vi "IMAQdx_AbsImage_Flea3_v4.7.vi"() -> ()   [LabVIEW 2013] (continued)
0\tVimaging\t0\t0\t1\t0\t1\t1\t0\tbMOTpow(0.5)\tProbePow\t0\tXshimrMOT\tYshimrMOT\tZshimVar\tODTpowZ(DipPowZ)\tVimaging\t0\t0\tHimaging\t0\t0\t0\t0\t0\t0\t0\t0\t0\t0\t0\t0\t0\t0\trMOTdelta(-(rMOTstirDetI +stirWidthF/2))\tODTpowBlue(0)\tODTpowXY(DipPowCr)\tvarWaveP2\tProbePow2\tAmp688(depumpPow)\trMOTpow3\tODTpowX(DipPowX2)\tfreq\tHeatingAmp\t0\tSine\tDetuning\tsingleFreqDet +20\tDoppCoolDet-DoppCoolSweep\tdopCoolT*1000\tDetuning\tsingleFreqStirDet + 20\tsingleFreqStirDet + SFramp + SFramp2\tloadT*1000\tBlueBN\tBlueLaserProbeBN\tSSteckBN\tShortSteckDDS\tPixisPos(TOF)\tCycle Wait for Move\t0\t0\t0\t0\t0\t0\t0\t0\t0\t0\t0\t0\t0\t0\t0\t0\t0\t0\t0\t0\t0\t0\t0\t0\r\narm DIP FLEA\t\tRamp\t1\tcameraArmT\t0\t0\t0\t0\t0\t0\t0\t0\t0\t0\t0\t0\t0\t0\t0\t0\t0\t0\t0\t0\t0\t0\t0\t0\t0\t1\t1\t0\t0\t0\t1\t0\t0\tplus_zman\tminus_zman\tcompensation\trMOTcurrF\trMOTpow3\tcombAmplitude(combWidthF)\trMOTdelta(-(rMOTbroadDetuningF +combWidthF/2))\tODTpowHLat(DipPowHLat)\t0\tVimaging\t0\t0\t0\t0\t1\t0\t0\tbMOTpow(0.5)\tProbePow\t0\tXshimrMOT\tYshimrMOT\tZshimVar\tODTpowZ(DipPowZ3)\tVimaging\t0\t0\tHimaging\t0\t0\t0\t0\t0\t0\t0\t0\t0\t0\t0\t0\t0\t0\trMOTdelta(-(rMOTstirDetI +stirWidthF/2))\tODTpowBlue(0)\tODTpowXY(DipPowCrTOF)\tvarWaveP1\tProbePow2\tAmp688(depumpPow)\trMOTpow3\tODTpowX(DipPowXTOF)\tfreq\tHeatingAmp\t0\tSine\tDetuning\tsingleFreqDet +20\tDoppCoolDet-DoppCoolSweep\tdopCoolT*1000\tDetuning\tsingleFreqStirDet + 20\tsingleFreqStirDet + SFramp + SFramp2\tloadT*1000\tBlueBN\tBlueLaserProbeBN\tSSteckBN\tShortSteckDDS\tPixisPos(TOF)\tCycle Wait for Move\t0\t0\t0\t0\t0\t0\t0\t0\t0\t0\t0\t0\t0\t0\t0\t0\t0\t0\t0\t0\t0\t0\t0\t0\r\narm BEC FLEA\t\tRamp\t0\tcameraArmT\t1\t1\t1\t1\t1\t1\t0\t0\t0\t0\t0\t0\t0\t0\t0\t0\t0\t0\t0\t0\t0\t0\t0\t0\t0\t1\t1\t0\t0\t0\t1\t0\t0\tplus_zman\tminus_zman\tcompensation\trMOTcurrF\trMOTpow3\tcombAmplitude(combWidthF)\trMOTdelta(-(rMOTbroadDetuningF +combWidthF/2))\tODTpowHLat(DipPowHLat)\t0\tVimaging\t0\t0\t0\t0\t1\t0\t0\tbMOTpow(0.5)\tProbePow\t0\tXshimrMOT\tYshimrMOT\tZshimVar\tODTpowZ(DipPowZ3)\tVimaging\t0\t0\tHimaging\t0\t0\t0\t0\t0\t0\t0\t0\t0\t0\t0\t0\t0\t0\trMOTdelta(-(rMOTstirDetI +stirWidthF/2))\tODTpowBlue(BlueDipPow)\tExpFinal(tEvap1,ODTpowXY(DipPowCr2),ODTpowXY(DipPowCr3),tau)\tvarWaveP1\tProbePow2\tAmp688(depumpPow)\trMOTpow3\tExpFinal(tEvap1,ODTpowX(DipPowX2),ODTpowX(DipPowX3),tau)\tfreq\tHeatingAmp\t0\tSine\tDetuning\tsingleFreqDet +20\tDoppCoolDet-DoppCoolSweep\tdopCoolT*1000\tDetuning\tsingleFreqStirDet + 20\tsingleFreqStirDet + SFramp + SFramp2\tloadT*1000\tBlueBN\tBlueLaserProbeBN\tSSteckBN\tShortSteckDDS\tPixisPos(TOF)\tCycle Wait for Move\t0\t0\t0\t0\t0\t0\t0\t0\t0\t0\t0\t0\t0\t0\t0\t0\t0\t0\t0\t0\t0\t0\t0\t0\r\natom img\t\tRamp\t1\texposureT\t0\t0\t0\t0\t0\t0\t0\t0\t1\t0\t0\t0\t0\t1\t0\t0\t0\t0\t1\t0\t0\t0\t0\t0\t0\t1\t1\t0\t0\t0\t1\t0\t0\tplus_zman\tminus_zman\tcompensation\trMOTcurrF\trMOTpow3\tcombAmplitude(combWidthF)\trMOTdelta(-(rMOTbroadDetuningF +combWidthF/2))\tODTpowHLat(DipPowHLat)\t0\tVimaging\t0\t0\t0\t0\t0\t0\t0\tbMOTpow(0.5)\tProbePow\t0\tXshimrMOT\tYshimrMOT\tZshimVar\tODTpowZ(DipPowZ)\tVimaging\t0\t0\tHimaging\t0\t0\t0\t0\t0\t0\t0\t0\t0\t0\t0\t0\t0\t0\trMOTdelta(-(rMOTstirDetI +stirWidthF/2))\tODTpowBlue(BlueDipPow)\tODTpowXY(DipPowCr)\tvarWaveP1\tProbePow2\tAmp688(depumpPow)\trMOTpow3\tODTpowX(DipPowX)\tfreq\tHeatingAmp\t0\tSine\tDetuning\tsingleFreqDet +20\tDoppCoolDet-DoppCoolSweep\tdopCoolT*1000\tDetuning\tsingleFreqStirDet + 20\tsingleFreqStirDet + SFramp + SFramp2\tloadT*1000\tBlueBN\tBlueLaserProbeBN\tSSteckBN\tShortSteckDDS\tPixisPos(TOF)\tCycle Wait for Move\t0\t0\t0\t0\t0\t0\t0\t0\t0\t0\t0\t0\t0\t0\t0\t0\t0\t0\t0\t0\t0\t0\t0\t0\r\natom img\t\tRamp\t0\t2.8e-3\t0\t0\t0\t0\t0\t0\t0\t0\t0\t1\t0\t0\t0\t0\t0\t0\t0\t0\t0\t0\t0\t0\t0\t0\t0\t1\t1\t0\t0\t0\t1\t1\t0\tplus_zman\tminus_zman\tcompensation\trMOTcurrF\trMOTpow3\tcombAmplitude(combWidthF)\trMOTdelta(-(rMOTbroadDetuningF +combWidthF/2))\tODTpowHLat(DipPowHLat)\t0\tVimaging\t0\t0\t1\t0\t1\t1\t0\tbMOTpow(0.5)\tProbePow\t0\tXshimrMOT\tYshimrMOT\tZshimVar\tODTpowZ(DipPowZ)\tVimaging\t0\t0\tHimaging\t0\t0\t0\t0\t0\t0\t0\t0\t0\t0\t0\t0\t0\t0\trMOTdelta(-(rMOTstirDetI +stirWidthF/2))\tODTpowBlue(0)\tODTpowXY(DipPowCr)\tvarWaveP2\tProbePow2\tAmp688(depumpPow)\trMOTpow3\tODTpowX(DipPowX)\tfreq\tHeatingAmp\t0\tSine\tDetuning\tsingleFreqDet +20\tDoppCoolDet-DoppCoolSweep\tdopCoolT*1000\tDetuning\tsingleFreqStirDet + 20\tsingleFreqStirDet + SFramp + SFramp2\tloadT*1000\tBlueBN\tBlueLaserProbeBN\tSSteckBN\tShortSteckDDS\tPixisPos(TOF)\tCycle Wait for Move\t0\t0\t0\t0\t0\t0\t0\t0\t0\t0\t0\t0\t0\t0\t0\t0\t0\t0\t0\t0\t0\t0\t0\t0\r\ntransmit img\t\tRamp\t1\t.7\t0\t0\t0\t0\t0\t0\t0\t0\t0\t1\t0\t0\t0\t0\t0\t0\t0\t0\t0\t0\t0\t0\t0\t0\t0\t1\t1\t0\t0\t0\t1\t1\t0\tplus_zman\tminus_zman\tcompensation\trMOTcurrF\trMOTpow3\tcombAmplitude(combWidthF)\trMOTdelta(-(rMOTbroadDetuningF +combWidthF/2))\tODTpowHLat(DipPowHLat)\t0\tVimaging\t0\t0\t1\t0\t1\t1\t0\tbMOTpow(0.5)\tProbePow\t0\tXshimrMOT\tYshimrMOT\tZshimVar\tODTpowZ(DipPowZ)\tVimaging\t0\t0\t0\t0\t1\t0\t0\t0\t0\t0\t0\t0\t0\t0\t0\t0\t0\trMOTdelta(-(rMOTstirDetI +stirWidthF/2))\tODTpowBlue(0)\tODTpowXY(DipPowCr)\tvarWaveP2\tProbePow2\tAmp688(depumpPow)\trMOTpow3\tODTpowX(DipPowX)\tfreq\tHeatingAmp\t0\tSine\tDetuning\tsingleFreqDet +20\tDoppCoolDet-DoppCoolSweep\tdopCoolT*1000\tDetuning\tsingleFreqStirDet + 20\tsingleFreqStirDet + SFramp + SFramp2\tloadT*1000\tBlueBN\tBlueLaserProbeBN\tSSteckBN\tShortSteckDDS\tPixisPos(TOF)\tCycle Wait for Move\t0\t0\t0\t0\t0\t0\t0\t0\t0\t0\t0\t0\t0\t0\t0\t0\t0\t0\t0\t0\t0\t0\t0\t0\r\narm PIXIS\t\tRamp\t0\t.007\t0\t0\t0\t0\t0\t0\t0\t0\t0\t1\t1\t0\t0\t0\t1\t1\t0\t0\t0\t0\t0\t0\t0\t0\t0\t1\t1\t0\t0\t0\t1\t1\t0\tplus_zman\tminus_zman\tcompensation\trMOTcurrF\trMOTpow1\tcombAmplitude(combWidthF)\trMOTdelta(-(rMOTbroadDetuningF +combWidthF/2))\tODTpowHLat(DipPowHLat)\t0\tVimaging\t0\t0\t1\t0\t1\t1\t0\tbMOTpow(0.5)\tProbePow\t0\tXshimrMOT\tYshimrMOT\tZshimVar\tODTpowZ(DipPowZ)\tVimaging\t0\t0\t0\t0\t1\t0\t0\t0\t0\t0\t0\t0\t0\t0\t0\t0\t0\trMOTdelta(-(rMOTstirDetI +stirWidthF/2))\tODTpowBlue(0)\tODTpowXY(DipPowCr)\tvarWaveP2\tProbePow2\tAmp688(depumpPow)\trMOTpow1\tODTpowX(DipPowX)\tfreq\tHeatingAmp\t0\tSine\tDetuning\tsingleFreqDet +20\tDoppCoolDet-DoppCoolSweep\tdopCoolT*1000\tDetuning\tsingleFreqStirDet + 20\tsingleFreqStirDet + SFramp + SFramp2\tloadT*1000\tBlueBN\tBlueLaserProbeBN\tSSteckBN\tShortSteckDDS\tPixisPos(TOF)\tCycle Wait for Move\t0\t0\t0\t0\t0\t0\t0\t0\t0\t0\t0\t0\t0\t0\t0\t0\t0\t0\t0\t0\t0\t0\t0\t0\r\narm FLEA\t\tRamp\t1\tcameraArmT\t0\t0\t0\t0\t0\t0\t0\t0\t0\t1\t1\t0\t0\t0\t1\t1\t0\t0\t0\t0\t0\t0\t0\t0\t0\t1\t1\t0\t0\t0\t1\t0\t0\tplus_zman\tminus_zman\tcompensation\trMOTcurrF\trMOTpow1\tcombAmplitude(combWidthF)\trMOTdelta(-(rMOTbroadDetuningF +combWidthF/2))\tODTpowHLat(DipPowHLat)\t0\tVimaging\t0\t0\t0\t0\t1\t0\t0\tbMOTpow(0.5)\tProbePow\t0\tXshimrMOT\tYshimrMOT\tZshimVar\tODTpowZ(DipPowZ)\tVimaging\t0\t0\t0\t0\t1\t0\t0\t0\t0\t0\t0\t0\t0\t0\t0\t0\t0\trMOTdelta(-(rMOTstirDetI +stirWidthF/2))\tODTpowBlue(0)\tODTpowXY(DipPowCr)\tvarWaveP2\tProbePow2\tAmp688(depumpPow)\trMOTpow1\tODTpowX(DipPowX)\tfreq\tHeatingAmp\t0\tSine\tDetuning\tsingleFreqDet +20\tDoppCoolDet-DoppCoolSweep\tdopCoolT*1000\tDetuning\tsingleFreqStirDet + 20\tsingleFreqStirDet + SFramp + SFramp2\tloadT*1000\tBlueBN\tBlueLaserProbeBN\tSSteckBN\tShortSteckDDS\tPixisPos(TOF)\tCycle Wait for Move\t0\t0\t0\t0\t0\t0\t0\t0\t0\t0\t0\t0\t0\t0\t0\t0\t0\t0\t0\t0\t0\t0\t0\t0\r\nprobe img\t\tRamp\t1\texposureT\t0\t0\t0\t0\t0\t0\t0\t0\t1\t1\t1\t0\t0\t1\t1\t1\t0\t0\t0\t0\t0\t0\t0\t0\t0\t1\t1\t0\t0\t0\t1\t0\t0\tplus_zman\tminus_zman\tcompensation\trMOTcurrF\trMOTpow1\tcombAmplitude(combWidthF)\trMOTdelta(-(rMOTbroadDetuningF +combWidthF/2))\tODTpowHLat(DipPowHLat)\t0\tVimaging\t0\t0\t0\t0\t0\t0\t0\tbMOTpow(0.5)\tProbePow\t0\tXshimrMOT\tYshimrMOT\tZshimVar\tODTpowZ(DipPowZ)\tVimaging\t0\t0\t0\t0\t1\t0\t0\t0\t0\t0\t0\t0\t0\t0\t0\t0\t0\trMOTdelta(-(rMOTstirDetI +stirWidthF/2))\tODTpowBlue(0)\tODTpowXY(DipPowCr)\tvarWaveP2\tProbePow2\tAmp688(depumpPow)\trMOTpow1\tODTpowX(DipPowX)\tfreq\tHeatingAmp\t0\tSine\tDetuning\tsingleFreqDet +20\tDoppCoolDet-DoppCoolSweep\tdopCoolT*1000\tDetuning\tsingleFreqStirDet + 20\tsingleFreqStirDet + SFramp + SFramp2\tloadT*1000\tBlueBN\tBlueLaserProbeBN\tSSteckBN\tShortSteckDDS\tPixisPos(TOF)\tCycle Wait for Move\t0\t0\t0\t0\t0\t0\t0\t0\t0\t0\t0\t0\t0\t0\t0\t0\t0\t0\t0\t0\t0\t0\t0\t0\r\nprobe img\t\tRamp\t0\t2.8e-3\t0\t0\t0\t0\t0\t0\t0\t0\t0\t1\t1\t0\t0\t0\t1\t1\t0\t0\t0\t0\t0\t0\t0\t0\t0\t1\t1\t0\t0\t0\t1\t1\t0\tplus_zman\tminus_zman\tcompensation\trMOTcurrF\trMOTpow1\tcombAmplitude(combWidthF)\trMOTdelta(-(rMOTbroadDetuningF +combWidthF/2))\tODTpowHLat(DipPowHLat)\t0\tVimaging\t0\t0\t1\t0\t1\t1\t0\tbMOTpow(0.5)\tProbePow\t0\tXshimrMOT\tYshimrMOT\tZshimVar\tODTpowZ(DipPowZ)\tVimaging\t0\t0\t0\t0\t1\t0\t0\t0\t0\t0\t0\t0\t0\t0\t0\t0\t0\trMOTdelta(-(rMOTstirDetI +stirWidthF/2))\tODTpowBlue(0)\tODTpowXY(DipPowCr)\tvarWaveP2\tProbePow2\tAmp688(depumpPow)\trMOTpow1\tODTpowX(DipPowX)\tfreq\tHeatingAmp\t0\tSine\tDetuning\tsingleFreqDet +20\tDoppCoolDet-DoppCoolSweep\tdopCoolT*1000\tDetuning\tsingleFreqStirDet + 20\tsingleFreqStirDet + SFramp + SFramp2\tloadT*1000\tBlueBN\tBlueLaserProbeBN\tSSteckBN\tShortSteckDDS\tPixisPos(TOF)\tCycle Wait for Move\t0\t0\t0\t0\t0\t0\t0\t0\t0\t0\t0\t0\t0\t0\t0\t0\t0\t0\t0\t0\t0\t0\t0\t0\r\ntransmit img\t\tRamp\t1\t.600\t0\t0\t0\t0\t0\t0\t0\t0\t0\t1\t1\t0\t0\t0\t1\t1\t0\t0\t0\t0\t0\t0\t0\t0\t0\t1\t1\t0\t0\t0\t1\t1\t0\tplus_zman\tminus_zman\tcompensation\trMOTcurrF\trMOTpow1\tcombAmplitude(combWidthF)\trMOTdelta(-(rMOTbroadDetuningF +combWidthF/2))\tODTpowHLat(DipPowHLat)\t0\tVimaging\t0\t0\t1\t0\t1\t1\t0\tbMOTpow(0.5)\tProbePow\t0\tXshimrMOT\tYshimrMOT\tZshimVar\tODTpowZ(DipPowZ)\tVimaging\t0\t0\t0\t0\t1\t0\t0\t0\t0\t0\t0\t0\t0\t0\t0\t0\t0\trMOTdelta(-(rMOTstirDetI +stirWidthF/2))\tODTpowBlue(0)\tODTpowXY(DipPowCr)\tvarWaveP2\tProbePow2\tAmp688(depumpPow)\trMOTpow1\tODTpowX(DipPowX)\tfreq\tHeatingAmp\t0\tSine\tDetuning\tsingleFreqDet +20\tDoppCoolDet-DoppCoolSweep\tdopCoolT*1000\tDetuning\tsingleFreqStirDet + 20\tsingleFreqStirDet + SFramp + SFramp2\tloadT*1000\tBlueBN\tBlueLaserProbeBN\tSSteckBN\tShortSteckDDS\tPixisPos(TOF)\tCycle Wait for Move\t0\t0\t0\t0\t0\t0\t0\t0\t0\t0\t0\t0\t0\t0\t0\t0\t0\t0\t0\t0\t0\t0\t0\t0\r\ntransmit img\t\tRamp\t1\t.025\t0\t0\t0\t0\t0\t0\t0\t0\t0\t1\t1\t0\t0\t0\t1\t1\t0\t0\t0\t0\t0\t0\t0\t0\t0\t1\t1\t0\t0\t0\t1\t1\t0\tplus_zman\tminus_zman\tcompensation\trMOTcurrF\trMOTpow1\tcombAmplitude(combWidthF)\trMOTdelta(-(rMOTbroadDetuningF +combWidthF/2))\tODTpowHLat(DipPowHLat2)\t0\tVimaging\t0\t0\t1\t0\t1\t1\t0\tbMOTpow(0.5)\tProbePow\t0\tXshimrMOT\tYshimrMOT\tZshimVar\tODTpowZ(DipPowZ)\tVimaging\t0\t0\t0\t0\t1\t0\t0\t0\t0\t0\t0\t0\t0\t0\t0\t0\t0\trMOTdelta(-(rMOTstirDetI +stirWidthF/2))\tODTpowBlue(.05)\tODTpowXY(DipPowCr)\tvarWaveP2\tProbePow2\tAmp688(depumpPow)\trMOTpow1\tODTpowX(DipPowX)\tfreq\tHeatingAmp\t0\tSine\tDetuning\tsingleFreqDet +20\tDoppCoolDet-DoppCoolSweep\tdopCoolT*1000\tDetuning\tsingleFreqStirDet + 20\tsingleFreqStirDet + SFramp + SFramp2\tloadT*1000\tBlueBN\tBlueLaserProbeBN\tSSteckBN\tShortSteckDDS\tPixisPos(TOF)\tCycle Wait for Move\t0\t0\t0\t0\t0\t0\t0\t0\t0\t0\t0\t0\t0\t0\t0\t0\t0\t0\t0\t0\t0\t0\t0\t0\r\narm PIXIS\t\tRamp\t0\t.007\t0\t0\t0\t0\t0\t0\t0\t0\t0\t1\t1\t0\t0\t0\t1\t1\t0\t0\t0\t0\t0\t0\t0\t0\t0\t1\t1\t0\t0\t0\t1\t0\t0\tplus_zman\tminus_zman\tcompensation\trMOTcurrF\trMOTpow1\tcombAmplitude(combWidthF)\trMOTdelta(-(rMOTbroadDetuningF +combWidthF/2))\tODTpowHLat(DipPowHLat2)\t0\tVimaging\t0\t0\t0\t0\t1\t1\t0\tbMOTpow(0.5)\tProbePow\t0\tXshimrMOT\tYshimrMOT\tZshimVar\tODTpowZ(DipPowZ)\tVimaging\t0\t0\t0\t0\t1\t0\t0\t0\t0\t0\t0\t0\t0\t0\t0\t0\t0\trMOTdelta(-(rMOTstirDetI +stirWidthF/2))\tODTpowBlue(0)\tODTpowXY(DipPowCr)\tvarWaveP2\tProbePow2\tAmp688(depumpPow)\trMOTpow1\tODTpowX(DipPowX)\tfreq\tHeatingAmp\t0\tSine\tDetuning\tsingleFreqDet +20\tDoppCoolDet-DoppCoolSweep\tdopCoolT*1000\tDetuning\tsingleFreqStirDet + 20\tsingleFreqStirDet + SFramp + SFramp2\tloadT*1000\tBlueBN\tBlueLaserProbeBN\tSSteckBN\tShortSteckDDS\tPixisPos(TOF)\tCycle Wait for Move\t0\t0\t0\t0\t0\t0\t0\t0\t0\t0\t0\t0\t0\t0\t0\t0\t0\t0\t0\t0\t0\t0\t0\t0\r\narm FLEA\t\tRamp\t1\tcameraArmT\t0\t0\t0\t0\t0\t0\t0\t0\t0\t1\t1\t0\t0\t0\t1\t1\t0\t0\t0\t0\t0\t0\t0\t0\t0\t1\t1\t0\t0\t0\t1\t0\t0\tplus_zman\tminus_zman\tcompensation\trMOTcurrF\trMOTpow1\tcombAmplitude(combWidthF)\trMOTdelta(-(rMOTbroadDetuningF +combWidthF/2))\tODTpowHLat(DipPowHLat2)\t0\tVimaging\t0\t0\t0\t0\t1\t0\t0\tbMOTpow(0.5)\tProbePow\t0\tXshimrMOT\tYshimrMOT\tZshimVar\tODTpowZ(DipPowZ)\tVimaging\t0\t0\t0\t0\t1\t0\t0\t0\t0\t0\t0\t0\t0\t0\t0\t0\t0\trMOTdelta(-(rMOTstirDetI +stirWidthF/2))\tODTpowBlue(.05)\tODTpowXY(DipPowCr)\tvarWaveP2\tProbePow2\tAmp688(depumpPow)\trMOTpow1\tODTpowX(DipPowX)\tfreq\tHeatingAmp\t0\tSine\tDetuning\tsingleFreqDet +20\tDoppCoolDet-DoppCoolSweep\tdopCoolT*1000\tDetuning\tsingleFreqStirDet + 20\tsingleFreqStirDet + SFramp + SFramp2\tloadT*1000\tBlueBN\tBlueLaserProbeBN\tSSteckBN\tShortSteckDDS\tPixisPos(TOF)\tCycle Wait for Move\t0\t0\t0\t0\t0\t0\t0\t0\t0\t0\t0\t0\t0\t0\t0\t0\t0\t0\t0\t0\t0\t0\t0\t0\r\nbg img\t\tRamp\t1\texposureT\t0\t0\t0\t0\t0\t0\t0\t0\t0\t1\t1\t0\t0\t0\t1\t1\t0\t0\t0\t0\t0\t0\t0\t0\t0\t1\t1\t0\t0\t0\t1\t0\t0\tplus_zman\tminus_zman\tcompensation\trMOTcurrF\trMOTpow1\tcombAmplitude(combWidthF)\trMOTdelta(-(rMOTbroadDetuningF +combWidthF/2))\tODTpowHLat(DipPowHLat2)\t0\tVimaging\t0\t0\t0\t0\t0\t0\t0\tbMOTpow(0.5)\tProbePow\t0\tXshimrMOT\tYshimrMOT\tZshimVar\tODTpowZ(DipPowZ)\tVimaging\t0\t0\t0\t0\t1\t0\t0\t0\t0\t0\t0\t0\t0\t0\t0\t0\t0\trMOTdelta(-(rMOTstirDetI +stirWidthF/2))\tODTpowBlue(.05)\tODTpowXY(DipPowCr)\tvarWaveP2\tProbePow2\tAmp688(depumpPow)\trMOTpow1\tODTpowX(DipPowX)\tfreq\tHeatingAmp\t0\tSine\tDetuning\tsingleFreqDet +20\tDoppCoolDet-DoppCoolSweep\tdopCoolT*1000\tDetuning\tsingleFreqStirDet + 20\tsingleFreqStirDet + SFramp + SFramp2\tloadT*1000\tBlueBN\tBlueLaserProbeBN\tSSteckBN\tShortSteckDDS\tPixisPos(TOF)\tCycle Wait for Move\t0\t0\t0\t0\t0\t0\t0\t0\t0\t0\t0\t0\t0\t0\t0\t0\t0\t0\t0\t0\t0\t0\t0\t0\r\nbg img\t\tRamp\t0\t1e-4\t0\t0\t0\t0\t0\t0\t0\t0\t0\t1\t1\t0\t0\t0\t1\t1\t0\t0\t0\t0\t0\t0\t0\t0\t0\t1\t1\t0\t0\t0\t1\t1\t0\tplus_zman\tminus_zman\tcompensation\trMOTcurrF\trMOTpow1\tcombAmplitude(combWidthF)\trMOTdelta(-(rMOTbroadDetuningF +combWidthF/2))\tODTpowHLat(DipPowHLat)\t0\tVimaging\t0\t0\t1\t0\t1\t1\t0\tbMOTpow(0.5)\tProbePow\t0\tXshimrMOT\tYshimrMOT\tZshimVar\tODTpowZ(DipPowZ)\tVimaging\t0\t0\t0\t0\t1\t0\t0\t0\t0\t0\t0\t0\t0\t0\t0\t0\t0\trMOTdelta(-(rMOTstirDetI +stirWidthF/2))\tODTpowBlue(0)\tODTpowXY(DipPowCr)\tvarWaveP2\tProbePow2\tAmp688(depumpPow)\trMOTpow1\tODTpowX(DipPowX)\tfreq\tHeatingAmp\t0\tSine\tDetuning\tsingleFreqDet +20\tDoppCoolDet-DoppCoolSweep\tdopCoolT*1000\tDetuning\tsingleFreqStirDet + 20\tsingleFreqStirDet + SFramp + SFramp2\tloadT*1000\tBlueBN\tBlueLaserProbeBN\tSSteckBN\tShortSteckDDS\tPixisPos(TOF)\tCycle Wait for Move\t0\t0\t0\t0\t0\t0\t0\t0\t0\t0\t0\t0\t0\t0\t0\t0\t0\t0\t0\t0\t0\t0\t0\t0\r\ntransmit img\t\tRamp\t1\t.625\t0\t0\t0\t0\t0\t0\t0\t1\t0\t1\t1\t0\t0\t0\t1\t1\t0\t0\t0\t0\t0\t0\t0\t0\t0\t1\t1\t0\t0\t0\t1\t1\t0\tplus_zman\tminus_zman\tcompensation\trMOTcurrF\trMOTpow1\tcombAmplitude(combWidthF)\trMOTdelta(-(rMOTbroadDetuningF +combWidthF/2))\tODTpowHLat(DipPowHLat)\t0\tVimaging\t0\t0\t1\t0\t1\t1\t0\tbMOTpow(0.5)\tProbePow\t0\tXshimrMOT\tYshimrMOT\tZshimVar\tODTpowZ(DipPowZ)\tVimaging\t0\t0\t0\t0\t1\t0\t0\t0\t0\t0\t0\t0\t0\t0\t0\t0\t0\trMOTdelta(-(rMOTstirDetI +stirWidthF/2))\tODTpowBlue(0)\tODTpowXY(DipPowCr)\tvarWaveP2\tProbePow2\tAmp688(depumpPow)\trMOTpow1\tODTpowX(DipPowX)\tfreq\tHeatingAmp\t0\tSine\tDetuning\tsingleFreqDet +20\tDoppCoolDet-DoppCoolSweep\tdopCoolT*1000\tDetuning\tsingleFreqStirDet + 20\tsingleFreqStirDet + SFramp + SFramp2\tloadT*1000\tBlueBN\tBlueLaserProbeBN\tSSteckBN\tShortSteckDDS\tPixisPos(TOF)\tCycle Wait for Move\t0\t0\t0\t0\t0\t0\t0\t0\t0\t0\t0\t0\t0\t0\t0\t0\t0\t0\t0\t0\t0\t0\t0\t0\r\nalignment\t\tRamp\t1\t.1\t1\t1\t1\t1\t1\t1\t1\t0\t1\t0\t1\t0\t1\t1\t1\t1\t0\t0\t0\t0\t0\t0\t0\t0\t1m\t1\t1\t0\t1\t0\t0\t1\t1\tplus_zman\tminus_zman\tcompensation\tMOTcurrent\trMOTpow1\tcombAmplitude(combWidthI)\trMOTdelta(-(rMOTbroadDetuningI +combWidthI/2))\tODTpowHLat(DipPowHLat2)\t1\t0\t1\t1\t1\t1\t1\t1\t0\tbMOTpow(MOTPow)\tProbePow\t0\tXshim\tYshim\tZshim\tODTpowZ(DipPowZ3)\t0\t1\t1\t0\t1\t1\t0\t1\t0\t0\t0\t0\t0\t0\t0\t0\t0\t0\trMOTdelta(-(rMOTstirDetI +stirWidthI/2))\tODTpowBlue(0.05)\tExpFinal(tEvap1,ODTpowXY(DipPowCr2),ODTpowXY(DipPowCr3),tau)\tvarWaveP2\tProbePow2\tAmp688(depumpPow)\trMOTpow3\tExpFinal(tEvap1,ODTpowX(DipPowX2),ODTpowX(DipPowX3),tau)\tfreq\tHeatingAmp\t0\tSine\tDetuning\tsingleFreqDet +20\tDoppCoolDet-DoppCoolSweep\tdopCoolT*1000\tDetuning\tsingleFreqStirDet + 20\tsingleFreqStirDet + SFramp + SFramp2\tloadT*1000\tBlueBN\tBlueLaserBeatnote\tSSteckBN\tShortSteckDDS\tPixisPos(TOF)\tCycle Wait for Move\t0\t0\t0\t0\t0\t0\t0\t0\t0\t0\t0\t0\t0\t0\t0\t0\t0\t0\t0\t0\t0\t0\t0\t0\r\n\r\n\r\n"
  in  "Source of Control Data":refnum<k21>="\\\\CONTROL\\VariableLibrary\\CycleDone"
  out "SPE delete path":path=path "C:/Users/Lab/Documents/LightField/LabviewTemp.spe"
  in  "Flea Data Series Name":string="Sr_Flea_Seq_4"
  in  "Camera Name":T2="GrassHp XZ"
  in  "Experiment":T3(ring)=enum."Sr"
  in  "Accept parameters from remote system":bool=TRUE
  in  "Flea Magnification":dbl=3.863
  in  "Flea Image direction":enum16{"XY", "XZ"}(ring)=enum."XZ"
  in  "Flea Imaging technique":enum16{"Absorption", "Fluorescence", "RawImage"}(ring)
  in  "Send Flea data to Igor?":bool=TRUE
  out "Command to Igor":string="AutoRunV3(\"Sr_Flea_Seq_4\",\"I:\\\\Data\\\\FL3_32S2Mtemp.ibw\") "